vi "caratterizzazione statica simulata.vi"() -> ()   [LabVIEW 2018]
uses:
  <vilib>/Analysis/baseanly.llb/Mean (DBL).vi
  <vilib>/Analysis/1siggen.llb/Ramp Pattern by Samples.vi
  <vilib>/Waveform/WDTFileIO.llb/Read Waveform from File.vi
  <vilib>/Analysis/NI_AALPro.lvlib
  <vilib>/Analysis/NI_AALBase.lvlib
panel:
  out "x-y":dbl[](array[numeric])
  out "INL %":dbl[](array[numeric])
  out "INL":dbl[](array[numeric])
  out "DNL":dbl[](array[numeric])
  out "LSB":dbl=0.1519775390625
  out "errore di guadagno":dbl=-0.034927520231509135
  out "errore di offset":dbl=-0.15564196553170906
  in  "stop":bool
  out "confonto":waveform(dbl)[](graph)=[{"t0"=timestamp(0 s since 1904-01-01), "dt"=0.004982701600323113, "Y"=array[248 elements]}, {"t0"=timestamp(0 s since 1904-01-01), "dt"=0.004982701600323113, "Y"=array[248 elements]}]
  out "intercept":dbl=-0.15564196553170906
  out "slope":dbl=0.9650724797684909
  out "indice di fine":i32[](array[numeric])=[10553, 14702, 18410, 24032, 29072, 33973, 38684, 43759, 48762, 53829, 58566, 63769, 68809, 73412, 78542, 83853, 88638, 93636, 98514, 103589, 108653, 113398, 118273, 123509, 128703, 133365, 138778, 143472, 148541, 153010, 158307, 163411, 167929, 173135, 178386, 182780, 188160, 193234, 197837, 202459, 207383, 212670, 217564, 222404, 227315, 232454, 237392, 242851, 247410, 252305, 256862, 262199, 266697, 271516, 276705, 281573, 286380, 291462, 296679, 301679, 306702, 311225, 316260, 321355, 326341, 331341, 336357, 341073, 345722, 350822, 356252, 360877, 365931, 371149, 375674, 380415, 385724, 390676, 395245, 401082, 405408, 409944, 415402, 419878, 424944, 430022, 435013, 440241, 444831, 450150, 455201, 459830, 464635, 467282, 472505, 477402, 482135, 487275, 492130, 496949, 502893, 507713, 512452, 517011, 522087, 527103, 532413, 536864, 541812, 547074, 551999, 556011, 562452, 566924, 571619, 576575, 581266, 587333, 591695, 596783, 601609, 606347, 610931, 616707, 620605, 624894, 629585, 635086, 639525, 645367, 649534, 654939, 659632, 665063, 669700, 675004, 679618, 684812, 689582, 694687, 699311, 704460, 709765, 714532, 719586, 724149, 729504, 734336, 739151, 744053, 749467, 754681, 759809, 764200, 769309, 774591, 778780, 783260, 788381, 794587, 798304, 804115, 808498, 813858, 818348, 823495, 828881, 833279, 838154, 843392, 847777, 852602, 857525, 862779, 867505, 872895, 877618, 882742, 887429, 892281, 897836, 902272, 907076, 912514, 918056, 922059, 926741, 932349, 936778, 941602, 946818, 951716, 956530, 961405, 966656, 971890, 976505, 981493, 986759, 991566, 996299, 1001887, 1006673, 1011668, 1016448, 1021168, 1026247, 1031413, 1037082, 1041527, 1045369, 1050447, 1055524, 1060718, 1065694, 1070498, 1075734, 1080795, 1085783, 1090759, 1095398, 1101034, 1105553, 1109937, 1115672, 1120527, 1125193, 1130625, 1135510, 1140428, 1145082, 1150538, 1155197, 1160002, 1165422, 1170299, 1175099, 1180158, 1185342, 1190074, 1195335, 1200386, 1205207, 1209885, 1214716, 1220118, 1225460, 1230049]
  out "min value":dbl=-19.53125
  out "max value":dbl=19.375
  out "caratteristica statica":cluster{dbl[], dbl[]}(graph)
  out "numeri di bit eq":dbl=8.0
  out "Mediane\n delle transizioni":dbl[](array[numeric])=[-19.39370584954765, -19.26486280487805, -19.15207654723127, -18.94002681518152, -18.81046195652174, -18.661694729136165, -18.45028409090909, -18.34582018927445, -18.201582136445243, -18.037142255892256, -17.949425795053003, -17.793135683760685, -17.517246136865342, -17.432795698924732, -17.270084566596193, -17.117346938775512, -16.952903682719548, -16.811532331511838, -16.64025907494145, -16.542604813664596, -16.32124042145594, -16.166721635883906, -16.033358895705522, -15.934488758029978, -15.716675588865096, -15.534143518518519, -15.36766353046595, -15.29296875, -15.11100113122172, -14.86298076923077, -14.77724032586558, -14.604229041916168, -14.524773316062177, -14.286583619702176, -14.165913200723327, -14.049651856763926, -13.853874063670412, -13.686899038461538, -13.462536196911197, -13.370367462311558, -13.23948598130841, -13.035689317673379, -12.94039080796253, -12.699593321917808, -12.537852112676056, -12.452281605113637, -12.280780663329162, -12.056744749596122, -11.961125753012048, -11.749188311688311, -11.648903145695364, -11.479233014861995, -11.297991071428571, -11.166015625, -11.010210396039604, -10.88365486257928, -10.744847670250897, -10.508199257425742, -10.334889481707316, -10.21445571192053, -10.020303672316384, -9.941689311594203, -9.806614349775785, -9.655842082860387, -9.37845515970516, -9.27115926157697, -9.187325418994414, -8.988413958641063, -8.856382978723405, -8.719416182170542, -8.4754873853211, -8.354021486643438, -8.256118881118882, -8.068374515503876, -7.955374513618677, -7.774051047120419, -7.565684713375796, -7.382258421985815, -7.228605388272583, -7.072415014164306, -6.948084677419355, -6.80516975308642, -6.648706896551724, -6.519293478260869, -6.330997242647059, -6.2238245118191164, -6.02729301948052, -5.875726744186046, -5.7252126963350785, -5.542534722222222, -5.391343390804598, -5.2892620894160585, -5.0262141280353205, -4.9504180960548885, -4.7640893734643734, -4.56, -4.4807785299806575, -4.277059037900875, -4.1823563664596275, -3.985247905027933, -3.8293192675159236, -3.6578237410071943, -3.5679517133956384, -3.388087606837607, -3.21393544935806, -3.072465728715729, -2.8859661697247705, -2.7535601265822787, -2.5714597902097904, -2.402470930232558, -2.2607600732600734, -2.1814437984496124, -1.9689002403846154, -1.8377786624203822, -1.6501966059602649, -1.4662418655097613, -1.3408221797323137, -1.1649469339622642, -1.0021053500660502, -0.8637366584564861, -0.7145522388059702, -0.5464352720450282, -0.3958333333333333, -0.22629310344827586, -0.0712189226519337, 0.09493403247631935, 0.19866071428571427, 0.4228583916083916, 0.533960027100271, 0.7049682395644283, 0.8742297535211268, 1.0406123481781377, 1.1661052894211577, 1.3135843848580442, 1.4876089324618735, 1.631533530571992, 1.7699505649717515, 1.909041394335512, 2.1446958812260535, 2.258627502634352, 2.4144665948275863, 2.56791483113069, 2.7522950201207244, 2.8631438442211055, 3.0373406193078325, 3.1944064551422318, 3.4162924151696608, 3.573325163398693, 3.6799172794117645, 3.8474264705882355, 4.006932218309859, 4.160121681415929, 4.34473079004329, 4.454501651982379, 4.587215909090909, 4.776605156723964, 4.968996062992126, 5.0485899390243905, 5.2038298872180455, 5.4399475870253164, 5.520833333333333, 5.762725515463917, 5.895917338709677, 6.065517912772585, 6.170316951566951, 6.331521739130435, 6.524972707423581, 6.688864834337349, 6.847368421052631, 6.9454596134786915, 7.124870867768595, 7.237633689839572, 7.44529282115869, 7.532118055555555, 7.75462962962963, 7.882952008928571, 8.059860354223433, 8.178697776280323, 8.371108058608058, 8.49080023364486, 8.686715949820789, 8.847246503496503, 8.962091023489933, 9.107967134416544, 9.35525092936803, 9.493885869565217, 9.575892857142858, 9.796851783060921, 9.949864665354331, 10.0234375, 10.235927152317881, 10.352668845315904, 10.577546296296296, 10.63508064516129, 10.85109819121447, 11.057764021479713, 11.159598214285714, 11.337872439478584, 11.5356529209622, 11.615887745974955, 11.805489543726235, 12.026041666666666, 12.09131006006006, 12.306299115913555, 12.449661726804123, 12.542183195592287, 12.739392201834862, 12.934954353932584, 13.121350364963504, 13.206018518518519, 13.33891369047619, 13.465444711538462, 13.624198717948717, 13.850761515601784, 14.007881637168142, 14.200487012987013, 14.3125, 14.436046511627907, 14.633501838235293, 14.786402925531915, 14.918793503480279, 15.116448326055313, 15.228189149560118, 15.395220588235293, 15.593314321926488, 15.735659246575343, 15.89853028503563, 15.978020055970148, 16.163832720588236, 16.367445054945055, 16.469166666666666, 16.664922248803826, 16.76464160839161, 16.911962365591396, 17.096603460972016, 17.261970029239766, 17.44140625, 17.552595208845208, 17.80626558603491, 17.86122803806735, 18.001453488372093, 18.17064606741573, 18.34726443768997, 18.51252158894646, 18.660189636752136, 18.851600985221676, 18.972772277227723, 19.095905172413794]
  out "indice di inizio":i32[](array[numeric])=[2484, 14292, 17796, 23426, 28842, 33290, 38464, 43442, 48205, 53235, 58283, 63301, 68356, 73040, 78069, 83510, 88285, 93087, 97660, 102945, 108392, 113019, 118110, 123042, 128236, 133095, 138220, 143096, 147878, 152750, 157816, 162576, 167736, 172262, 177833, 182403, 187092, 192714, 197319, 202061, 206848, 211776, 216710, 222112, 226960, 231750, 236593, 242232, 247078, 252074, 256560, 261728, 266417, 271276, 276099, 281100, 285822, 291260, 296351, 301075, 306171, 310949, 315368, 319593, 325934, 330542, 335641, 340396, 345017, 350306, 355816, 360016, 364787, 370633, 375160, 380224, 385096, 390112, 394614, 400376, 405284, 409134, 414648, 419303, 424400, 428076, 434397, 439768, 444067, 449610, 454331, 458734, 464182, 466699, 471691, 476652, 481618, 486932, 491808, 496233, 501323, 506879, 511489, 516543, 521386, 526410, 531541, 536469, 541097, 545999, 551453, 555882, 560996, 566139, 571015, 576114, 580743, 586273, 590938, 595565, 601274, 605814, 610811, 615895, 620243, 624155, 629165, 634371, 639156, 644265, 648966, 654198, 659131, 664112, 669241, 674497, 679087, 684353, 689060, 693738, 699079, 703779, 708771, 714134, 719037, 723692, 729003, 734030, 738743, 743543, 749183, 753551, 758885, 763746, 768759, 773602, 778145, 783096, 788115, 793323, 798031, 803339, 808374, 813537, 817997, 823311, 828423, 832615, 837679, 842383, 847535, 852415, 857128, 862239, 867262, 872447, 877251, 882000, 887156, 891853, 897557, 901986, 906480, 911837, 917249, 921829, 926440, 931676, 936270, 941322, 946516, 951257, 956395, 961157, 966269, 971052, 975945, 980956, 986177, 991007, 996036, 1001377, 1006340, 1011159, 1016060, 1020805, 1026138, 1031057, 1036397, 1041257, 1045117, 1049927, 1055329, 1060045, 1065468, 1070190, 1075294, 1080365, 1085647, 1090195, 1094967, 1100347, 1105212, 1109614, 1114883, 1119797, 1124772, 1130089, 1134966, 1139973, 1144707, 1150329, 1154625, 1159723, 1164743, 1169957, 1174819, 1179751, 1184941, 1189391, 1194991, 1200297, 1204878, 1209306, 1214248, 1219509, 1225157, 1229614]
  out "Voltage Output":dbl[](graph)
  in  "file path (dialog if empty)":path=path "C:/Users/anna/Desktop/alberto/landi/laboratorio/CaratterizzazioneStaticaADC/FormaDonda"
  out "dt":dbl=9.999999974752427e-07
  # "Caratterizzazione ADC"
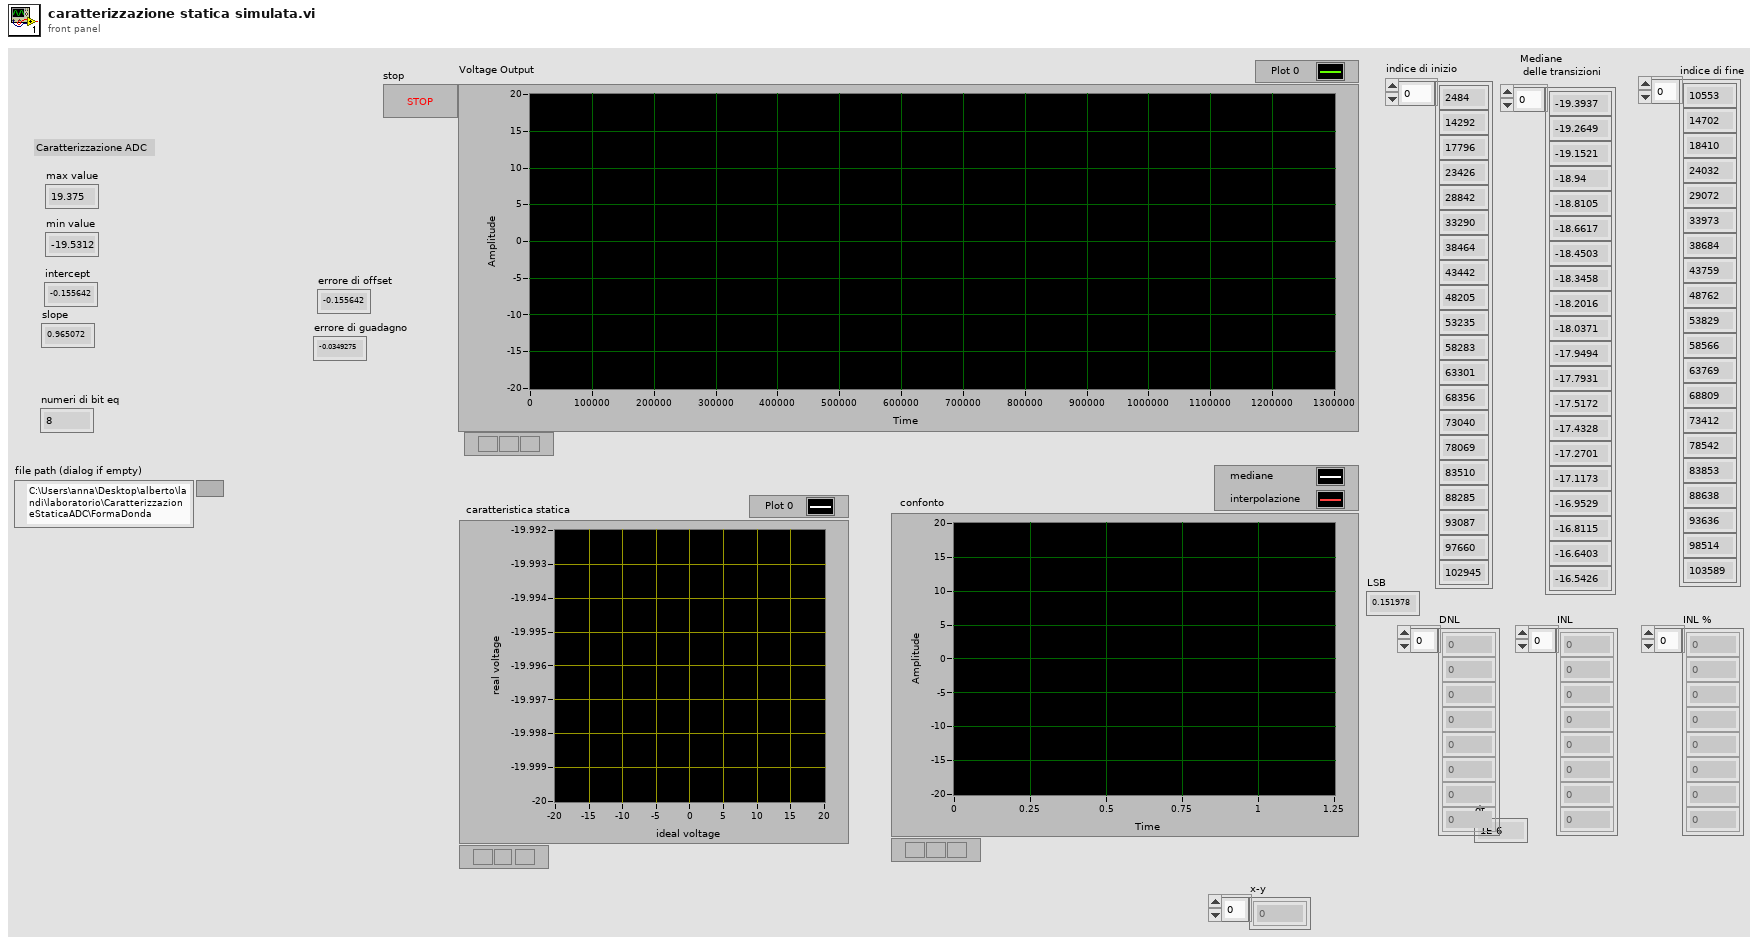
[diagram p1: front panel]
types:
  T1 = cluster{"Best Linear Fit":dbl[], "Ramp Pattern":dbl[]}
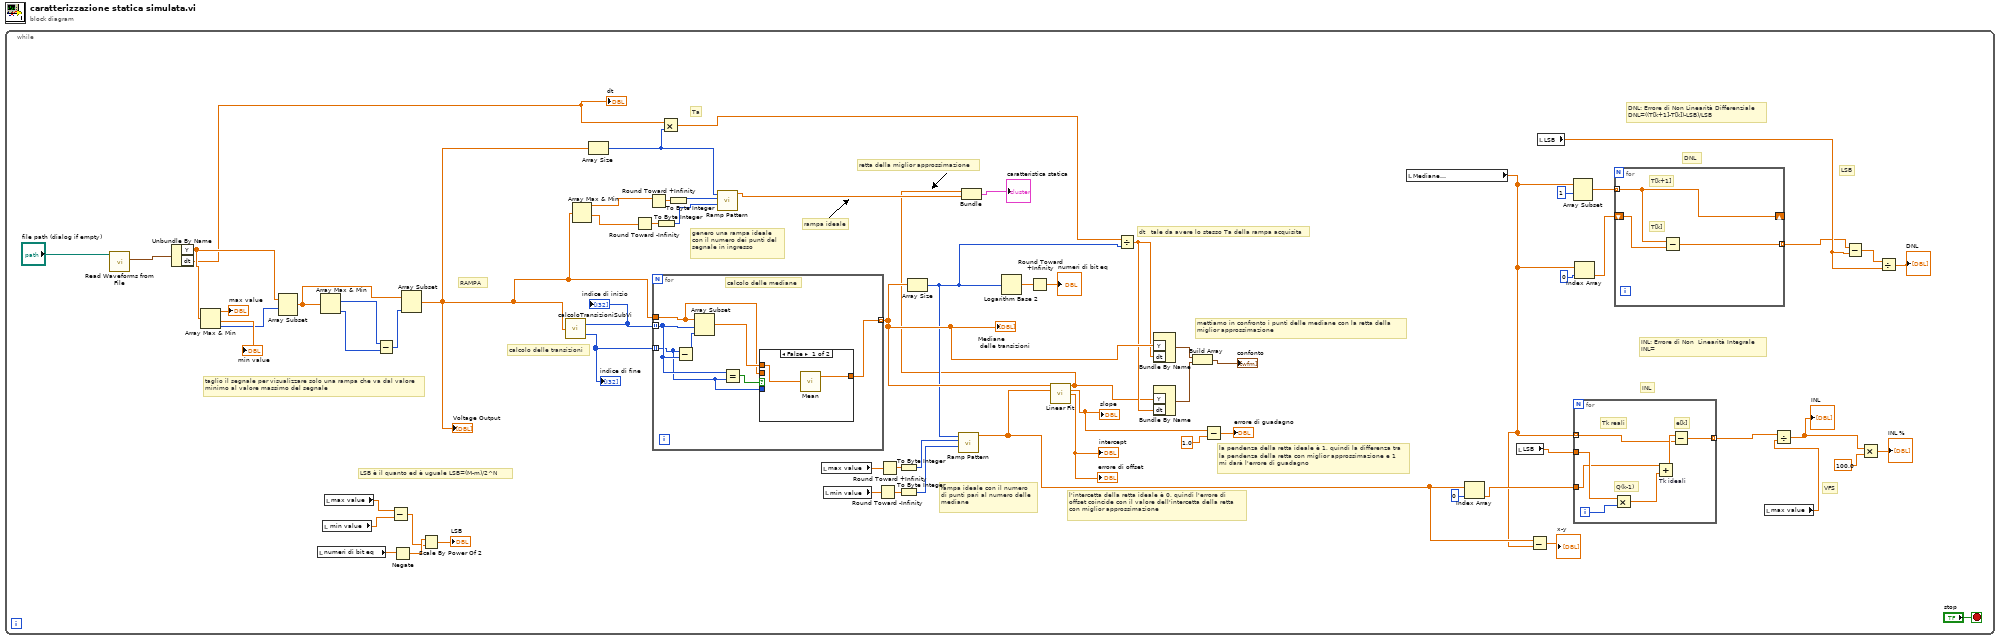
[diagram p0: block diagram]
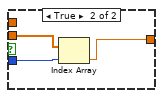
[diagram p2: hidden frame]
diagram:
  n1 = while {
    stop <- "stop" stop-if-true
    # "INL: Errore di Non  Linearità Integrale\nINL="
    # "DNL: Errore di Non Linearità Differenziale\nDNL=((T[k+1]-T[k])-LSB)/LSB"
    # "LSB è il quanto ed è uguale LSB=(M-m)/2^N"
    # "VFS"
    # "INL"
    # "LSB"
    # "DNL"
    # "rampa ideale con il numero\ndi punti pari al numero delle\nmediane"
    # "mettiamo in confronto i punti delle mediane con la retta della\nmiglior approssimazione"
    # "la pendenza della retta ideale è 1, quindi la differenza tra\nla pendenza della retta con miglior approssimazione e 1 \nmi darà l'errore di guadagno"
    # "l'intercetta della retta ideale è 0, quindi l'errore di \noffset coincide con il valore dell'intercetta della retta\ncon miglior approssimazione"
    # "rampa ideale"
    # "retta della miglior approssimazione"
    # "genero una rampa ideale\ncon il numero dei punti del\nsegnale in ingresso"
    # "RAMPA"
    # "taglio il segnale per visualizzare solo una rampa che va dal valore\nminimo al valore massimo del segnale"
    # "calcolo delle transizioni"
    # "dt   tale da avere lo stesso Ta della rampa acquisita"
    # "Ta"
    n2 = call-poly <vilib>:"Read Waveforms from File.vi"("file path (dialog if empty)"="file path (dialog if empty)") -> ("first waveform in record"=w52:waveform(dbl))  [unwired: 5 in, 3 out]
    n3 = Unbundle By Name(w52) -> ("Y"=w65:dbl[], "dt"=w50:dbl)
    "dt" <- w50
    n4 = Array Max & Min(array=w65) -> (max value=→"max value":dbl, min value=→"min value":dbl, min index (indices)=w60:i32)  [unwired: 1 out]
    n5 = Array Subset(array=w65, index=w60) -> (w56:dbl[])  [unwired: 1 in]
    n6 = local read "numeri di bit eq"() -> (w23:dbl)
    n7 = Array Max & Min(array=w56) -> (max index (indices)=w57:i32, min index (indices)=w58:i32)  [unwired: 2 out]
    n8 = local read "min value"() -> (w24:dbl)
    n9 = local read "max value"() -> (w25:dbl)
    n10 = Subtract(x=w57, y=w58) -> (x-y=w59:i32)
    n11 = Subtract(x=w25, y=w24) -> (x-y=w21:dbl)
    n12 = Negate(x=w23) -> (-x=w22:dbl)
    n13 = Array Subset(array=w56, length=w59) -> (w51:dbl[])  [unwired: 1 in]
    "Voltage Output" <- w51
    n14 = Scale By Power Of 2(n=w22, x=w21) -> (x*2^n=→"LSB":dbl)
    n15 = call "calcoloTransizioniSubVi.vi"("Array"=w51) -> ("indice di inizio"=w62:i32[], "indice di fine"=w61:i32[])
    "indice di inizio" <- w62
    "indice di fine" <- w61
    n16 = Array Max & Min(array=w51) -> (max value=w33:dbl, min value=w32:dbl)  [unwired: 2 out]
    n17 = Array Size(array=w51) -> (size(s)=w44:i32)
    n18 = Round Toward -Infinity(1:w32) -> (0:w34:dbl)
    n19 = Round Toward +Infinity(x=w33) -> (ceil(x): smallest int >= x=w35:dbl)
    n20 = for {
      tunnel: w51 -> [w82]
      tunnel: w62 -> [w81] mode=indexing
      tunnel: w61 -> [w80] mode=indexing
      tunnel: [w83] -> w48 mode=indexing
      # "calcolo delle mediane"
      n21 = Subtract(x=w80, y=w81) -> (x-y=w86:i32)
      n22 = Array Subset(array=w82, index=w81, length=w86) -> (w84:dbl[])
      n23 = Equal?(x=w81, y=w80) -> (x = y?=w85:bool)
      n24 = case shown="False" w85 {
        tunnel: w84 -> [w88 _]
        tunnel: [w87 w91] -> w83
        tunnel: w82 -> [_ w90]
        tunnel: w80 -> [_ w89]
        frame False {
          n25 = call-poly <vilib>:"Mean.vi"("X"=w88) -> ("mean"=w87:dbl)  [unwired: 1 out]
        }
        frame True {
          n26 = Index Array(array=w90, index=w89) -> (element=w91:dbl)
        }
      }
    }
    "Mediane\n delle transizioni" <- w48
    n27 = To Byte Integer(number=w34) -> (8bit integer=w30:i8)
    n28 = Multiply(x=w50, y=w44) -> (x*y=w49:dbl)
    n29 = To Byte Integer(number=w35) -> (8bit integer=w31:i8)
    n30 = call-poly <vilib>:"Ramp Pattern.vi"("start"=w30, "end"=w31, "samples"=w44) -> ("Ramp Pattern"=w43:dbl[])  [unwired: 7 in, 1 out]
    n31 = local read "max value"() -> (w42:dbl)
    n32 = local read "min value"() -> (w38:dbl)
    n33 = Round Toward -Infinity(1:w38) -> (0:w37:dbl)
    n34 = Round Toward +Infinity(x=w42) -> (ceil(x): smallest int >= x=w41:dbl)
    n35 = To Byte Integer(number=w41) -> (8bit integer=w40:i8)
    n36 = To Byte Integer(number=w37) -> (8bit integer=w39:i8)
    n37 = Array Size(array=w48) -> (size(s)=w47:i32)
    n38 = call-poly <vilib>:"Ramp Pattern.vi"("start"=w39, "end"=w40, "samples"=w47) -> ("Ramp Pattern"=w3:dbl[])  [unwired: 7 in, 1 out]
    n39 = Logarithm Base 2(1:w47) -> (0:w68:dbl)
    n40 = Round Toward +Infinity(x=w68) -> (ceil(x): smallest int >= x=→"numeri di bit eq":dbl)
    n41 = call <vilib>:"Linear Fit.vi"("Y"=w48, "X"=w3) -> ("Best Linear Fit"=w26:dbl[], "slope"=w29:dbl, "intercept"=→"intercept" →"errore di offset":dbl)  [unwired: 9 in, 2 out]
    "slope" <- w29
    n42 = Bundle("Best Linear Fit"=w26, "Ramp Pattern"=w43) -> (→"caratteristica statica":T1)  [unwired: 1 in]
    n43 = Divide(x=w49, y=w47) -> (x/y=w46:dbl)
    n44 = Bundle By Name("Y"=w48, "dt"=w46) -> (w54:waveform(dbl))  [unwired: 1 in]
    n45 = Bundle By Name("Y"=w26, "dt"=w46) -> (w45:waveform(dbl))  [unwired: 1 in]
    n46 = Build Array(w54, w45) -> (→"confonto":waveform(dbl)[])
    n47 = Subtract(x=w29, y=1.0) -> (x-y=→"errore di guadagno":dbl)
    n48 = local read "Mediane\n delle transizioni"() -> (w2:dbl[])
    n49 = Index Array(array=w3, index=0) -> (element=w9:dbl)
    n50 = local read "LSB"() -> (w11:dbl)
    n51 = Subtract(x=w3, y=w2) -> (x-y=→"x-y":dbl[])
    n52 = local read "LSB"() -> (w14:dbl)
    n53 = Array Subset(array=w2, index=1) -> (w17:dbl[])  [unwired: 1 in]
    n54 = for {
      tunnel: w9 -> [w73]
      tunnel: w2 -> [w70] mode=indexing
      tunnel: w11 -> [w75]
      tunnel: [w72] -> w4 mode=indexing
      i -> [w76]
      # "Tk reali"
      # "e[k]"
      # "Q(k-1)"
      n55 = Multiply(x=w75, y=w76) -> (x*y=w74:dbl)
      n56 = Add "Tk ideali"(x=w73, y=w74) -> (x+y=w71:dbl)
      n57 = Subtract(x=w71, y=w70) -> (x-y=w72:dbl)
    }
    n58 = Index Array(array=w2, index=0) -> (element=w15:dbl)
    n59 = for {
      tunnel: w17 -> [w79] mode=indexing
      shift-right: [w79] -> _
      shift-left: w15 -> [w78]
      tunnel: [w77] -> w5 mode=indexing
      # "T[k]"
      # "T[k+1]"
      n60 = Subtract(x=w79, y=w78) -> (x-y=w77:dbl)
    }
    n61 = local read "max value"() -> (w8:dbl)
    n62 = Divide(x=w4, y=w8) -> (x/y=w7:dbl[])
    "INL" <- w7
    n63 = Subtract(x=w5, y=w14) -> (x-y=w16:dbl[])
    n64 = Multiply(x=w7, y=100.0) -> (x*y=→"INL %":dbl[])
    n65 = Divide(x=w16, y=w14) -> (x/y=→"DNL":dbl[])
  }
